vi "Experiment_VSWR_MEASUREMENT.vi"() -> ()   [LabVIEW 2009]
uses:
  <vilib>/imath/engines/lvmath2/RunTimeEngine/ErrorHandling/NIMS_Finalize Error.vi
  <vilib>/imath/engines/lvmath2/RunTimeEngine/Parser/MC_Version.vi
  <vilib>/imath/engines/lvmath2/RunTimeEngine/NodeEndStatement/NIMS_NodeEndStatement_Output.vi
  <instcachedir>/0/NIMS_NodeEndStatement_Output_B70DDD75627E4997AAE11E9955EDAA25.lvgen/NIMS_NodeEndStatement_Output_B70DDD75627E4997AAE11E9955EDAA25_003.vi
  <instcachedir>/0/NIMS_NodeEndStatement_Output_B70DDD75627E4997AAE11E9955EDAA25.lvgen/NIMS_NodeEndStatement_Output_B70DDD75627E4997AAE11E9955EDAA25_002.vi
  <vilib>/imath/engines/lvmath/Functions/Error Handling/MergeErrorsWrapper.vi
  <instcachedir>/0/NIMS_NodeEndStatement_Output_B70DDD75627E4997AAE11E9955EDAA25.lvgen/NIMS_NodeEndStatement_Output_B70DDD75627E4997AAE11E9955EDAA25_000.vi
  <vilib>/imath/engines/lvmath2/RunTimeEngine/Managers/WorkSpace/UID Generator.vi
  <vilib>/imath/engines/lvmath/Functions/Error Handling/error.ctl
  <instcachedir>/0/NIMS_NodeEndStatement_Output_B70DDD75627E4997AAE11E9955EDAA25.lvgen/NIMS_NodeEndStatement_Output_B70DDD75627E4997AAE11E9955EDAA25_001.vi
  <vilib>/imath/engines/lvmath2/RunTimeEngine/Managers/SymbolTable/Clear UID.vi
  <vilib>/imath/engines/lvmath2/RunTimeEngine/VariableToken/NIMS_VariableToken_CondDefined.vi
  <instcachedir>/0/NIMS_VariableToken_CondDefined_5641E79000FB4D628475532441475385.lvgen/NIMS_VariableToken_CondDefined_5641E79000FB4D628475532441475385_002.vi
  <vilib>/imath/engines/lvmath/Functions/Error Handling/MC_Mask_Errors.vi
  <vilib>/imath/engines/lvmath2/RunTimeEngine/BuiltInFunctions/rem/NIMS_rem_no checks.vi
  <instcachedir>/0/NIMS_rem_no checks_4CC9B305AB7E42EF90AFC4973FB32F8D.lvgen/NIMS_rem_no checks_4CC9B305AB7E42EF90AFC4973FB32F8D_000.vi
  <vilib>/imath/engines/lvmath2/RunTimeEngine/BuiltInFunctions/uint32/NIMS_uint32(real).vi
  <instcachedir>/0/NIMS_uint32(real)_FDC83D68D45943DDB8F3F934FF8A712F.lvgen/NIMS_uint32(real)_FDC83D68D45943DDB8F3F934FF8A712F_000.vi
  <vilib>/imath/engines/lvmath2/RunTimeEngine/BuiltInFunctions/double/NIMS_double.vi
  <instcachedir>/0/NIMS_double_2CE444F3CE4146B199A482FE12545E45.lvgen/NIMS_double_2CE444F3CE4146B199A482FE12545E45_000.vi
  <vilib>/imath/engines/lvmath2/RunTimeEngine/RangeToken/NIMS_Range.vi
  <instcachedir>/0/NIMS_Range_6D647EC16A744C98B5DE1D649A2D648D.lvgen/NIMS_Range_6D647EC16A744C98B5DE1D649A2D648D_001.vi
  <vilib>/imath/engines/lvmath2/RunTimeEngine/BuiltInFunctions/length/NIMS_length(GV).vi
  <instcachedir>/0/NIMS_length(GV)_7D6E94E728E145E68721C53861296D96.lvgen/NIMS_length(GV)_7D6E94E728E145E68721C53861296D96_000.vi
  <instcachedir>/0/NIMS_Range_6D647EC16A744C98B5DE1D649A2D648D.lvgen/NIMS_Range_6D647EC16A744C98B5DE1D649A2D648D_000.vi
  <vilib>/imathl/engines/lvmath/Functions/Error Handling/Create Error.vi
  <vilib>/imath/engines/lvmath2/RunTimeEngine/ReplaceToken/NIMS_Replace - V(S)=S.vi
  <instcachedir>/0/NIMS_Replace - V(S)=S_670A9E0533664C1D848C8E58B3321B6A.lvgen/NIMS_Replace - V(S)=S_670A9E0533664C1D848C8E58B3321B6A_001.vi
  <vilib>/imath/engines/lvmath2/RunTimeEngine/ReplaceToken/NIMS_Replace - Size Check _(_)=S.vi
  <instcachedir>/0/NIMS_Replace - Size Check _(_)=S_8596181D73404097BAB9CBB006194BB0.lvgen/NIMS_Replace - Size Check _(_)=S_8596181D73404097BAB9CBB006194BB0_002.vi
  <vilib>/imath/engines/lvmath2/RunTimeEngine/ReplaceToken/NIMS_Replace - Check Linear.vi
  <instcachedir>/0/NIMS_Replace - Check Linear_9243CBB174894FF6977027453DA6955E.lvgen/NIMS_Replace - Check Linear_9243CBB174894FF6977027453DA6955E_002.vi
  <vilib>/imath/engines/lvmath2/RunTimeEngine/VariableToken/NIMS_VariableToken_CondDefinedDefinedByReplace.vi
  <instcachedir>/0/NIMS_VariableToken_CondDefinedDefinedByReplace_D162CFFC24174562A9FEA619A91E1A56.lvgen/NIMS_VariableToken_CondDefinedDefinedByReplace_D162CFFC24174562A9FEA619A91E1A56_002.vi
  <vilib>/imath/engines/lvmath2/RunTimeEngine/CommandStatement/MC_CommandStatement_break.vi
  <vilib>/imath/engines/lvmath2/RunTimeEngine/LocalVariableDefStatement/MC_LocalVariableDefStatement_Display.vi
  <vilib>/imath/engines/lvmath2/RunTimeEngine/RunTimeType/NIMS_RunTimeType_From StrictType (excl LVString).vi
  <vilib>/imath/engines/lvmath2/RunTimeEngine/ArithmeticOperatorToken/NIMS_ArithmeticOperator_times.vi
  <instcachedir>/0/NIMS_ArithmeticOperator_times_3987BC660D7947CD8628C10658A43225.lvgen/NIMS_ArithmeticOperator_times_3987BC660D7947CD8628C10658A43225_001.vi
  <instcachedir>/0/NIMS_ArithmeticOperator_times_3987BC660D7947CD8628C10658A43225.lvgen/NIMS_ArithmeticOperator_times_3987BC660D7947CD8628C10658A43225_000.vi
  <vilib>/imath/engines/lvmath2/RunTimeEngine/VariableToken/Read/NIMS_Get Elements - RV(_) - Check.vi
  <instcachedir>/0/NIMS_Get Elements - RV(_) - Check_60F12861D0564803969A5D0D0D1716CD.lvgen/NIMS_Get Elements - RV(_) - Check_60F12861D0564803969A5D0D0D1716CD_001.vi
  <instcachedir>/0/NIMS_VariableToken_CondDefined_5641E79000FB4D628475532441475385.lvgen/NIMS_VariableToken_CondDefined_5641E79000FB4D628475532441475385_001.vi
  <instcachedir>/0/NIMS_VariableToken_CondDefined_5641E79000FB4D628475532441475385.lvgen/NIMS_VariableToken_CondDefined_5641E79000FB4D628475532441475385_003.vi
  <vilib>/imath/engines/lvmath2/RunTimeEngine/BuiltInFunctions/abs/NIMS_abs(signed).vi
  <instcachedir>/0/NIMS_abs(signed)_C4FCB8E6058B49B797C7C8D53CA5F6EC.lvgen/NIMS_abs(signed)_C4FCB8E6058B49B797C7C8D53CA5F6EC_000.vi
  <instcachedir>/0/NIMS_Replace - V(S)=S_670A9E0533664C1D848C8E58B3321B6A.lvgen/NIMS_Replace - V(S)=S_670A9E0533664C1D848C8E58B3321B6A_000.vi
  <instcachedir>/0/NIMS_Replace - Size Check _(_)=S_8596181D73404097BAB9CBB006194BB0.lvgen/NIMS_Replace - Size Check _(_)=S_8596181D73404097BAB9CBB006194BB0_001.vi
  <instcachedir>/0/NIMS_Replace - Check Linear_9243CBB174894FF6977027453DA6955E.lvgen/NIMS_Replace - Check Linear_9243CBB174894FF6977027453DA6955E_001.vi
  <instcachedir>/0/NIMS_VariableToken_CondDefinedDefinedByReplace_D162CFFC24174562A9FEA619A91E1A56.lvgen/NIMS_VariableToken_CondDefinedDefinedByReplace_D162CFFC24174562A9FEA619A91E1A56_001.vi
  <instcachedir>/0/NIMS_Replace - V(S)=S_670A9E0533664C1D848C8E58B3321B6A.lvgen/NIMS_Replace - V(S)=S_670A9E0533664C1D848C8E58B3321B6A_002.vi
  <instcachedir>/0/NIMS_Replace - Size Check _(_)=S_8596181D73404097BAB9CBB006194BB0.lvgen/NIMS_Replace - Size Check _(_)=S_8596181D73404097BAB9CBB006194BB0_003.vi
  <instcachedir>/0/NIMS_Replace - Check Linear_9243CBB174894FF6977027453DA6955E.lvgen/NIMS_Replace - Check Linear_9243CBB174894FF6977027453DA6955E_003.vi
  <instcachedir>/0/NIMS_VariableToken_CondDefinedDefinedByReplace_D162CFFC24174562A9FEA619A91E1A56.lvgen/NIMS_VariableToken_CondDefinedDefinedByReplace_D162CFFC24174562A9FEA619A91E1A56_003.vi
  <vilib>/imath/engines/lvmath2/RunTimeEngine/Managers/SymbolTable/NIMS_WorkSpace.lvlib
panel:
  out "error out":errorcluster
  in  "2.TECNIQUE USED TO CALCULATE VSWR":bool
  out "error out":errorcluster
  in  "1.TECNIQUE USED TO CALCULATE VSWR":bool
  out "?":errorcluster
  out "?":errorcluster
  in  "?":T1(tab)
  out "?":dbl[](graph)
  out "Characteristic Impedance":dbl
  out "Voltage":dbl
  out "Distance(Meter)":dbl
  in  "Slide":dbl(slide) scale=0.0..0.3
  out "?":errorcluster
  in  "HELP FOR SLOTTED LINE":bool
  out "error out":errorcluster
  out "?":dbl[](graph)
  out "VSWR Meter":dbl(knob) caption="Meter" scale=500.0..1.0 scale format="%#_10g"
  out "Ideal VSWR":dbl
  in  "?":enum32{"LOADS"}(tab)
  in  "Type of Loads":T2(radio)
  out "Resistance":dbl
  out "Reactance":dbl
  in  "Resistance":dbl(slide) scale=0.0..1000.0
  in  "Reactance":dbl(slide) scale=0.0..1000.0
  out "?":errorcluster
  in  "HELP FOR LOADS":bool
  out "error out":errorcluster
  in  "?":enum32{"ATTENUATOR"}(tab)
  out "?":dbl[](graph)
  in  "Set the value of attenuation in dB":dbl(slide) scale=0.0..100.0
  out "?":errorcluster
  in  "HELP FOR ATTENUATOR":bool
  out "error out":errorcluster
  in  "?":enum32{"ISOLATOR"}(tab)
  out "?":dbl[](graph)
  in  "?":bool
  out "?":errorcluster
  in  "HELP FOR ISOLATOR":bool
  out "error out":errorcluster
  in  "?":enum32{"MODULATOR"}(tab)
  in  "Modulating Frequency(KHz)":dbl(slide) scale=0.5..1.5
  out "?":errorcluster
  out "?":dbl[](graph)
  in  "HELP FOR MODULATOR":bool
  out "error out":errorcluster
  in  "?":enum32{"SOURCE"}(tab)
  out "?":dbl[](graph)
  in  "Frequency of carrier wave(GHz)":dbl(slide) scale=8.0..15.0
  in  "Voltage":dbl(knob) scale=0.0..20.0 scale format="%#_10g"
  out "?":errorcluster
  in  "HELP FOR SOURCE":bool
  out "error out":errorcluster
  # "Slotted Line"
  # "Source"
  # "Variable Attenuator"
  # "Coaxial to rectangular adapter"
  # "Variable load"
  # "Connecting waveguide"
  # "Connecting waveguide"
  # "Connecting waveguide"
  # "Isolator"
  # "Matched load"
  # "VSWR Meter"
  # "Backward Direction"
  # "Forward direction"
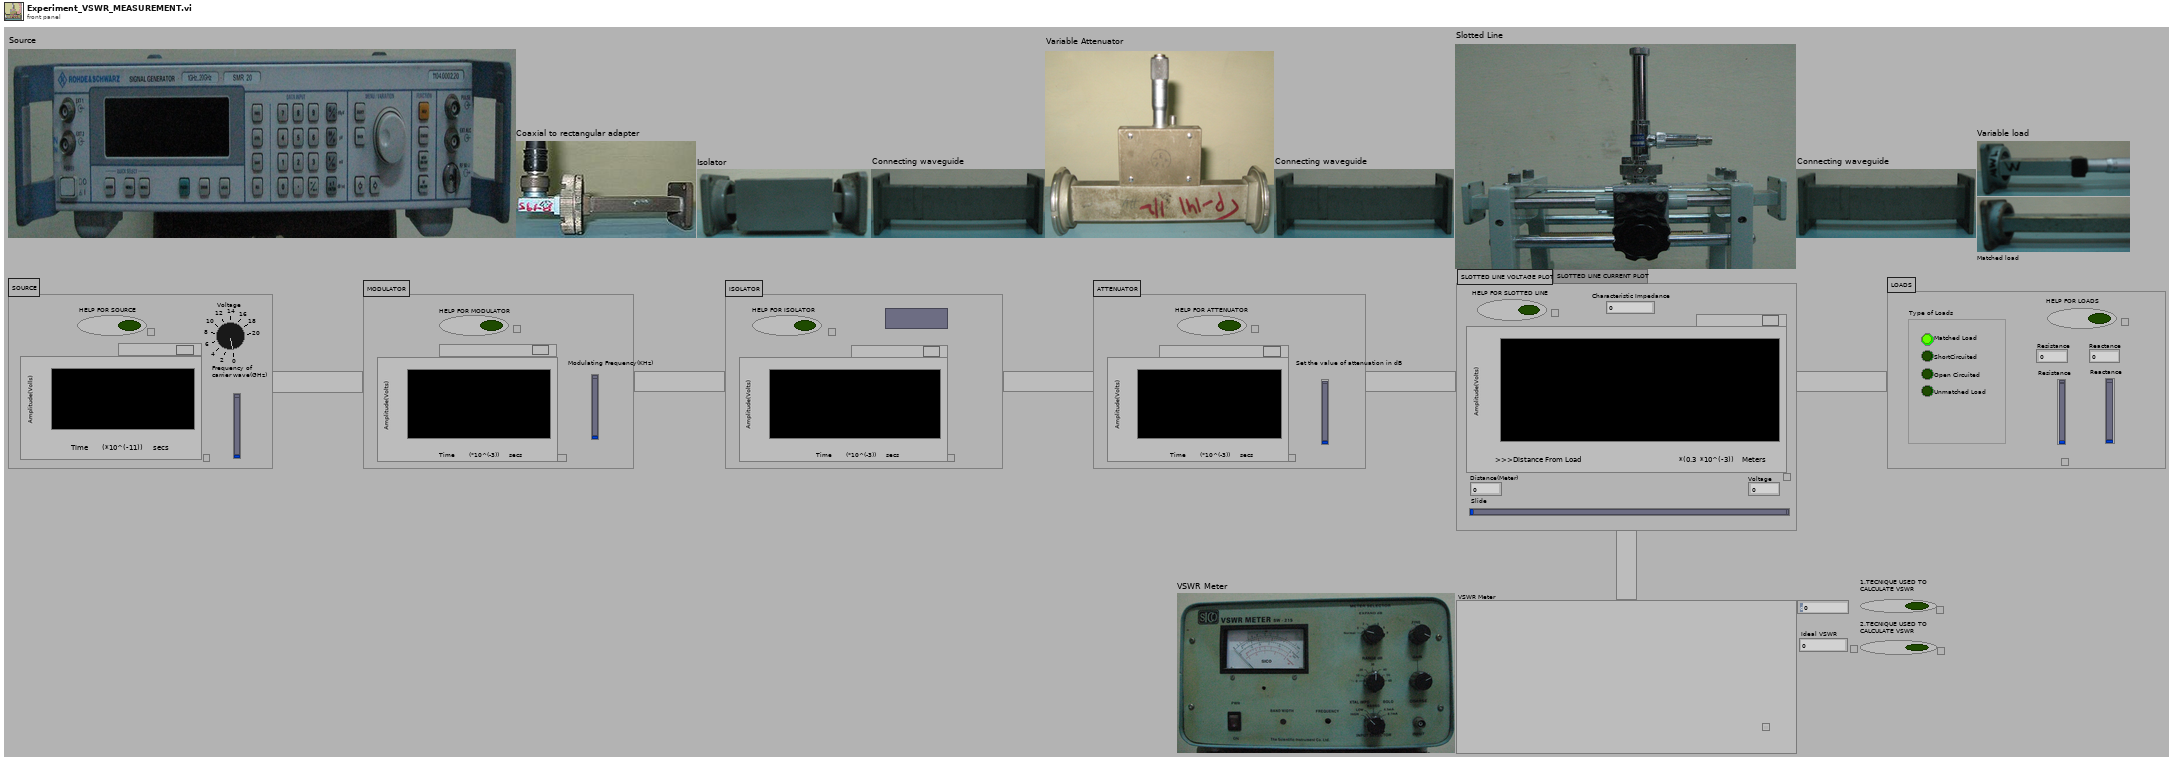
[diagram p1: front panel]
types:
  T1 = enum32{"SLOTTED LINE VOLTAGE PLOT", "SLOTTED LINE CURRENT PLOT"}
  T2 = enum32{"Matched Load", "ShortCircuited", "Open Circuited", "Unmatched Load"}
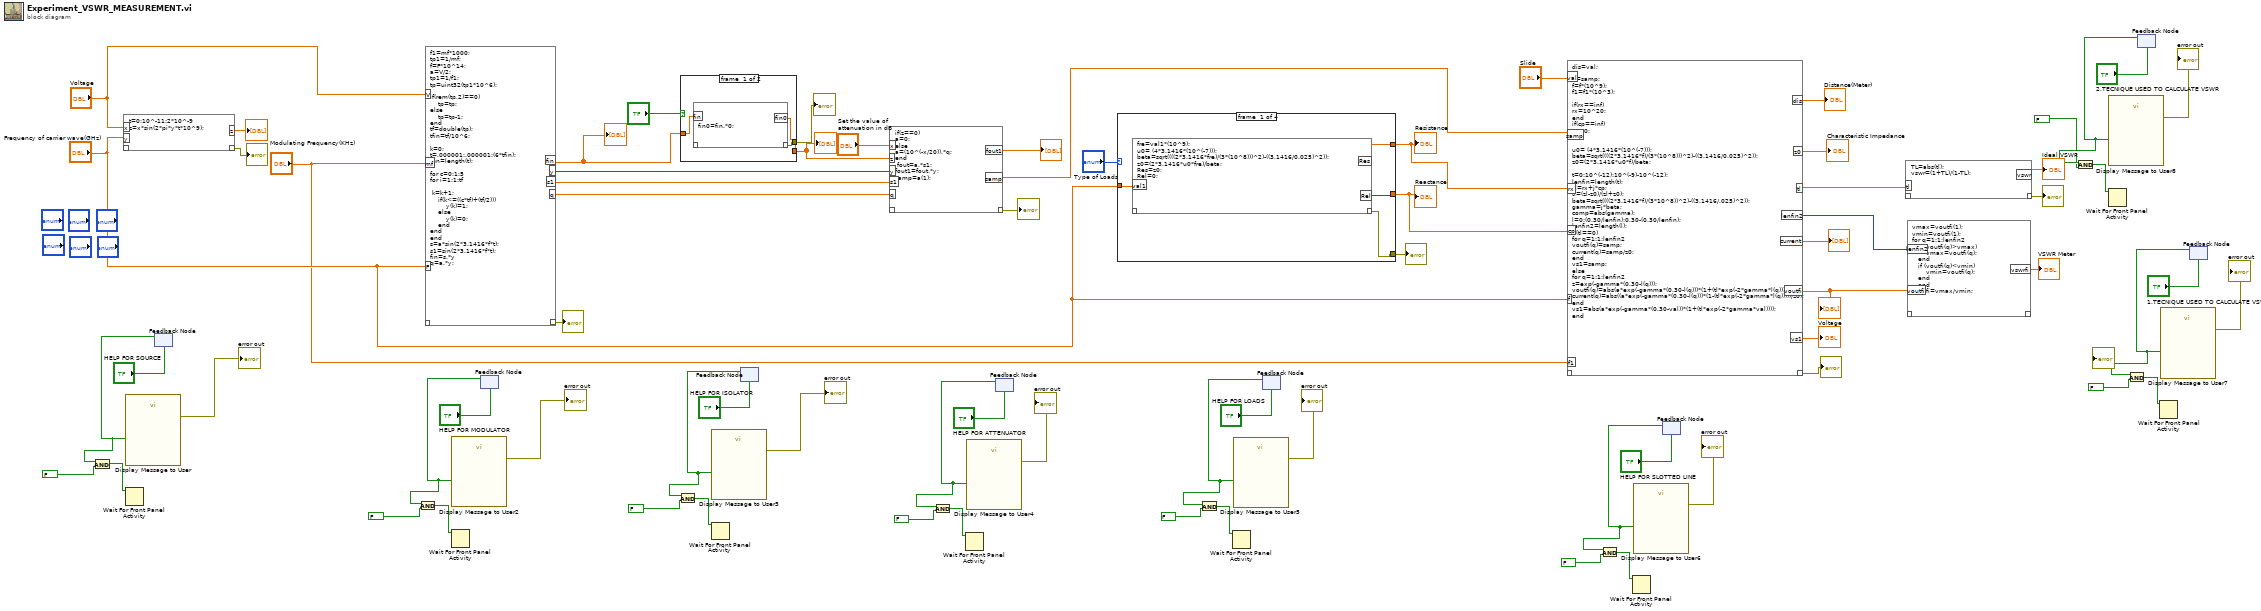
[diagram p0: block diagram]
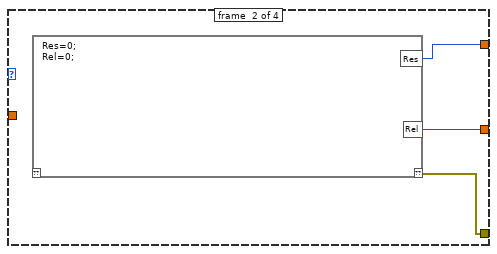
[diagram p2: hidden frame]
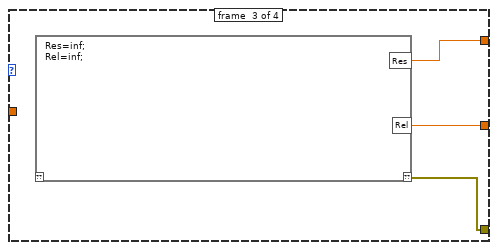
[diagram p3: hidden frame]
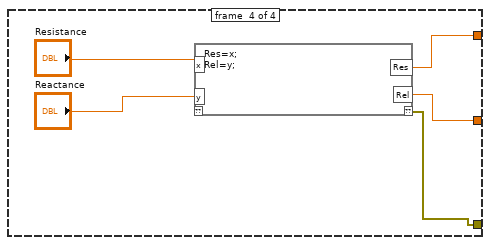
[diagram p4: hidden frame]
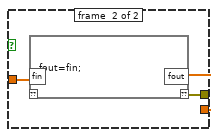
[diagram p5: hidden frame]
diagram:
  n1 = mathscript code="t=0:10^-11:2*10^-9\nz=x*sin(2*pi*y*t*10^9);"("x"="Voltage", "y"="Frequency of carrier wave(GHz)") -> ("??"=→"?":errorcluster, "z"=→"?":dbl[])  [unwired: 1 in]
  n2 = feedback #1("HELP FOR SOURCE") -> (w76:bool)
  n3 = And(x=w76, y=FALSE) -> (x .and. y?=w74:bool)
  n4 = Wait For Front Panel Activity(3:w74) -> ()  [unwired: 3 out]
  n5 = call "Display Message to User"("Enable"=w76) -> ("error out"=→"error out":errorcluster, "CLOSE"=w78:bool)  [unwired: 2 in, 7 out]
  n6 = mathscript code="f1=mf*1000;\ntp1=1/mf;\nf=F*10^14;\na=V/2;\ntp1=1/f1;\ntp=uint32(tp1*10^6);\n\nif(rem(tp,2)==0)\n    tp=tp;\nelse\n    tp=tp-1;\nend\ntf=double(tp);\ntfin=tf/10^6;\n\nk=0;\nt=.000001:.000001:(6*tfin);\nlen=length(t);\n\nfor c=0:1:5\nfor i=1:1:tf\n  \n k=k+1;\n    if(k<=((c*tf)+(tf/2)))\n        y(k)=1;\n    else\n        y(k)=0;\n    end\nend\nend\ns=a*sin(2*3.1416*f*t);\ns1=sin(2*3.1416*f*t);\nfin=s.*y\nq=a.*y;"("V"="Voltage", "mf"="Modulating Frequency(KHz)", "F"="Frequency of carrier wave(GHz)") -> ("??"=→"?":errorcluster, "fin"=w28:dbl[], "s1"=w23:dbl[], "q"=w22:dbl[], "y"=w24:i32[])  [unwired: 1 in]
  "?" <- w28
  n7 = feedback #2("HELP FOR MODULATOR") -> (w70:bool)
  n8 = And(x=w70, y=FALSE) -> (x .and. y?=w68:bool)
  n9 = Wait For Front Panel Activity(3:w68) -> ()  [unwired: 3 out]
  n10 = call "Display Message to User2"("Enable"=w70) -> ("error out"=→"error out":errorcluster, "CLOSE"=w72:bool)  [unwired: 2 in, 7 out]
  n11 = case shown="False" "?" {
    tunnel: [w83 w104] -> w25
    tunnel: w28 -> [w84 w105]
    tunnel: [w82 w103] -> w2
    frame #0 {
      n12 = mathscript code="fin0=fin.*0;"("fin"=w84) -> ("??"=w82:errorcluster, "fin0"=w83:dbl[])  [unwired: 1 in]
    }
    frame #1 {
      n13 = mathscript code="fout=fin;"("fin"=w105) -> ("??"=w103:errorcluster, "fout"=w104:dbl[])  [unwired: 1 in]
    }
  }
  "?" <- w25
  "?" <- w2
  n14 = feedback #3("HELP FOR ISOLATOR") -> (w64:bool)
  n15 = And(x=w64, y=FALSE) -> (x .and. y?=w62:bool)
  n16 = Wait For Front Panel Activity(3:w62) -> ()  [unwired: 3 out]
  n17 = call "Display Message to User3"("Enable"=w64) -> ("error out"=→"error out":errorcluster, "CLOSE"=w66:bool)  [unwired: 2 in, 7 out]
  n18 = mathscript code="if(z==0)\na=0; \nelse\na=(10^(-x/20)).*q;\nend\n fout=a.*s1;\nfout1=fout.*y;\nsamp=a(1);"("x"="Set the value of attenuation in dB", "z"=w25, "y"=w24, "s1"=w23, "q"=w22) -> ("??"=→"?":errorcluster, "fout1"=→"?":dbl[], "samp"=w17:dbl)  [unwired: 1 in]
  n19 = feedback #4("HELP FOR ATTENUATOR") -> (w58:bool)
  n20 = And(x=w58, y=FALSE) -> (x .and. y?=w56:bool)
  n21 = Wait For Front Panel Activity(3:w56) -> ()  [unwired: 3 out]
  n22 = call "Display Message to User4"("Enable"=w58) -> ("error out"=→"error out":errorcluster, "CLOSE"=w60:bool)  [unwired: 2 in, 7 out]
  n23 = case shown="\"Unmatched Load\"" "Type of Loads" {
    tunnel: "Frequency of carrier wave(GHz)" -> [w125 _ _ _]
    tunnel: [w123 w211 w237 w264] -> w16
    tunnel: [w124 w212 w238 w263] -> w15
    tunnel: [w122 w210 w236 w262] -> w1
    frame #0 {
      n24 = mathscript code="fre=val1*(10^9);\nu0= (4*3.1416*(10^(-7)));\nbeta=sqrt((((2*3.1416*fre)/(3*(10^8)))^2)-((3.1416/0.025)^2));\nz0=(2*3.1416*u0*fre)/beta;\nRes=z0;\nRel=0;"("val1"=w125) -> ("??"=w122:errorcluster, "Rel"=w124:i32, "Res"=w123:cdb)  [unwired: 1 in]
    }
    frame #1 {
      n25 = mathscript code="Res=0;\nRel=0;"() -> ("??"=w210:errorcluster, "Res"=w211:i32, "Rel"=w212:i32)  [unwired: 1 in]
    }
    frame #2 {
      n26 = mathscript code="Res=inf;\nRel=inf;"() -> ("??"=w236:errorcluster, "Res"=w237:dbl, "Rel"=w238:dbl)  [unwired: 1 in]
    }
    frame #3 {
      n27 = mathscript code="Res=x;\nRel=y;"("x"="Resistance", "y"="Reactance") -> ("??"=w262:errorcluster, "Res"=w264:dbl, "Rel"=w263:dbl)  [unwired: 1 in]
    }
  }
  "Resistance" <- w16
  "Reactance" <- w15
  "?" <- w1
  n28 = feedback #5("HELP FOR LOADS") -> (w52:bool)
  n29 = And(x=w52, y=FALSE) -> (x .and. y?=w50:bool)
  n30 = Wait For Front Panel Activity(3:w50) -> ()  [unwired: 3 out]
  n31 = call "Display Message to User5"("Enable"=w52) -> ("error out"=→"error out":errorcluster, "CLOSE"=w54:bool)  [unwired: 2 in, 7 out]
  n32 = mathscript code="dis=val;\n\na=samp;\nf=f*(10^9);\nf1=f1*(10^3);\n\nif(rx==inf)\nrx=10^20;\nend\nif(cp==inf)\ncp=0;\nend\n\nu0= (4*3.1416*(10^(-7)));\nbeta=sqrt((((2*3.1416*f)/(3*(10^8)))^2)-((3.1416/0.025)^2));\nz0=(2*3.1416*u0*f)/beta;\n\nt=0:10^(-12):10^(-9)-10^(-12);\nlenfin=length(t);\nzl=rx+j*cp;\ntl=(zl-z0)/(zl+z0);\nbeta=sqrt((((2*3.1416*f)/(3*10^8))^2)-((3.1416/.025)^2));\ngamma=j*beta;\ncomp=abs(gamma);\nl=0:(0.30/lenfin):0.30-(0.30/lenfin);\nlenfin2=length(l);\nif(tl==0)\nfor q=1:1:lenfin2\nvoutfi(q)=samp;\ncurrent(q)=samp/z0;\nend\nvs1=samp;\nelse\nfor q=1:1:lenfin2\nz=exp(-gamma*(0.30-l(q)));\nvoutfi(q)=abs(a*exp(-gamma*(0.30-l(q)))*(1+(tl*exp(-2*gamma*l(q)))));\ncurrent(q)=abs((a*exp(-gamma*(0.30-l(q)))*(1-(tl*exp(-2*gamma*l(q)))))/z0);\nend\nvs1=abs(a*exp(-gamma*(0.30-val))*(1+(tl*exp(-2*gamma*val))));\nend"("val"="Slide", "samp"=w17, "rx"=w16, "cp"=w15, "f"="Frequency of carrier wave(GHz)", "f1"="Modulating Frequency(KHz)") -> ("??"=→"?":errorcluster, "dis"=→"Distance(Meter)":dbl, "z0"=→"Characteristic Impedance":cdb, "tl"=w5:cdb, "lenfin2"=w10:i32, "current"=→"?":cdb[], "voutfi"=w8:dbl[], "vs1"=→"Voltage":dbl)  [unwired: 1 in]
  "?" <- w8
  n33 = feedback #6("HELP FOR SLOTTED LINE") -> (w46:bool)
  n34 = And(x=w46, y=FALSE) -> (x .and. y?=w44:bool)
  n35 = Wait For Front Panel Activity(3:w44) -> ()  [unwired: 3 out]
  n36 = call "Display Message to User6"("Enable"=w46) -> ("error out"=→"error out":errorcluster, "CLOSE"=w48:bool)  [unwired: 2 in, 7 out]
  n37 = mathscript code="TL=abs(tl);\nvswr=(1+TL)/(1-TL);"("tl"=w5) -> ("??"=→"?":errorcluster, "vswr"=→"Ideal VSWR":dbl)  [unwired: 1 in]
  n38 = mathscript code="vmax=voutfi(1);\nvmin=voutfi(1);\nfor q=1:1:lenfin2\n   if (voutfi(q)>vmax)\n       vmax=voutfi(q);\n   end\n   if (voutfi(q)<vmin)\n       vmin=voutfi(q);\n   end\n   end\nvswrfi=vmax/vmin;"("lenfin2"=w10, "voutfi"=w8) -> ("vswrfi"=→"VSWR Meter":dbl)  [unwired: 1 in, 1 out]
  n39 = feedback #7("2.TECNIQUE USED TO CALCULATE VSWR") -> (w34:bool)
  n40 = And(x=w34, y=FALSE) -> (x .and. y?=w32:bool)
  n41 = Wait For Front Panel Activity(3:w32) -> ()  [unwired: 3 out]
  n42 = call "Display Message to User8"("Enable"=w34) -> ("error out"=→"error out":errorcluster, "CLOSE"=w36:bool)  [unwired: 2 in, 7 out]
  n43 = feedback #8("1.TECNIQUE USED TO CALCULATE VSWR") -> (w40:bool)
  n44 = And(x=w40, y=FALSE) -> (x .and. y?=w38:bool)
  n45 = Wait For Front Panel Activity(3:w38) -> ()  [unwired: 3 out]
  n46 = call "Display Message to User7"("Enable"=w40) -> ("error out"=→"error out":errorcluster, "CLOSE"=w42:bool)  [unwired: 2 in, 7 out]
